vi "LOX_PID_screen_V2.5.vi"() -> ()   [LabVIEW 2022 SP3]
panel:
  out "Countdown Timer (CDT)":dbl format="T%<+%H:%M:%S%3u>t"
  out "Date":timestamp format="%<%d/%m/%Y>T"
  in  "Close":bool
  in  "Screen No":dbl
  out "Indian Standard Time (IST)":timestamp format="%<%H:%M:%S%2u>T"
  out "Boolean 77":bool
  out "B_GN_PV_01":bool caption="Boolean"
  out "Boolean 61":bool
  out "B_GN_PV_03":bool caption="Boolean"
  out "Boolean 76":bool
  out "B_GN_PV_04":bool caption="Boolean"
  out "Boolean 60":bool
  out "B_GN_PV_07":bool caption="Boolean"
  out "Boolean 73":bool
  out "B_LO_PV_02":bool caption="Boolean"
  out "B_GN_P_10":dbl format="%.2f bar"
  out "B_GN_P_09":dbl format="%.2f bar"
  out "B_GN_P_03":dbl format="%.2f bar"
  out "B_GN_CV_01":dbl format="%.0f %%"
  out "Boolean 59":bool
  out "B_GN_CV_01":bool caption="Boolean"
  out "B_GN_P_05":dbl format="%.2f bar"
  out "B_GN_P_04":dbl format="%.2f bar"
  out "B_GN_P_06":dbl format="%.2f bar"
  out "B_GN_P_32":dbl format="%.2f bar"
  out "Boolean 40":bool
  out "B_GN_PV_09":bool caption="Boolean"
  out "Boolean 41":bool
  out "B_GN_PV_08":bool caption="Boolean"
  out "B_GN_P_08":dbl format="%.2f bar"
  out "B_GN_P_07":dbl format="%.2f bar"
  out "B_GN_P_01":dbl format="%.2f bar"
  out "B_GO_P_04":dbl format="%.2f bar"
  out "B_GN_P_02":dbl format="%.2f bar"
  out "B_GN_P_12":dbl format="%.2f bar"
  out "B_GN_T_01":dbl format="%.2f bar"
  out "B_GN_P_11":dbl format="%.2f bar"
  out "B_GN_P_13":dbl format="%.2f bar"
  out "B_GO_P_03":dbl format="%.2f bar"
  out "B_GO_P_01":dbl format="%.2f bar"
  out "B_GO_P_02":dbl format="%.2f bar"
  out "B_GN_P_33":dbl format="%.2f bar"
  out "Boolean 74":bool
  out "B_LO_PV_09":bool caption="Boolean"
  out "Boolean 63":bool
  out "B_LO_PV":bool caption="Boolean"
  out "Boolean 66":bool
  out "B_LO_PV_13":bool caption="Boolean"
  out "Boolean 67":bool
  out "B_LO_PV_05":bool caption="Boolean"
  out "Boolean 65":bool
  out "B_LO_PV_06":bool caption="Boolean"
  out "B_LO_P_10":dbl format="%.2f bar"
  out "B_LO_FM_02":dbl format="%.2f Kg/s"
  out "Boolean 68":bool
  out "B_LO_PV_04":bool caption="Boolean"
  out "Boolean 75":bool
  out "B_LO_PV_12":bool caption="Boolean"
  out "Boolean 64":bool
  out "B_LO_PV_10":bool caption="Boolean"
  out "Boolean 62":bool
  out "B_LO_PV_11":bool caption="Boolean"
  out "B_LO_P_06":dbl format="%.2f bar"
  out "B_LO_T_06":dbl format="%.2f bar"
  out "Boolean 71":bool
  out "B_LO_PV_07":bool caption="Boolean"
  out "Boolean 69":bool
  out "B_LO_PV_08":bool caption="Boolean"
  out "B_LO_P_03":dbl format="%.2f bar"
  out "B_LO_T_03":dbl format="%.2f bar"
  out "B_LO_FM_03":dbl format="%.2f Kg/s"
  out "B_LO_P_09":dbl format="%.2f bar"
  out "Boolean 70":bool
  out "B_LO_PV_03":bool caption="Boolean"
  out "B_LO_P_08":dbl format="%.2f bar"
  out "B_LO_P_01":dbl format="%.2f bar"
  out "B_LO_T_01":dbl format="%.2f bar"
  out "Boolean 72":bool
  out "B_LO_PV_02":bool caption="Boolean"
  out "B_LO_P_02":dbl format="%.2f bar"
  out "B_LO_P_07":dbl format="%.2f bar"
  out "B_LO_T_02":dbl format="%.2f bar"
  out "B_LO_P_11":dbl format="%.2f bar"
  out "B_LN_T_03":dbl format="%.2f bar"
  out "B_LN_P_08":dbl format="%.2f bar"
  out "B_LO_P_05":dbl format="%.2f bar"
  out "B_LO_P_04":dbl format="%.2f bar"
  out "B_LO_T_04":dbl format="%.2f bar"
  out "B_LO_T_05":dbl format="%.2f bar"
  out "B_HE_P_03":dbl format="%.2f bar"
  out "B_HE_T_01":dbl format="%.2f bar"
  out "B_HE_P_04":dbl format="%.2f bar"
  out "B_HE_T_03":dbl format="%.2f bar"
  out "B_HE_T_02":dbl format="%.2f bar"
  out "B_HE_P_02":dbl format="%.2f bar"
  out "B_HE_P_01":dbl format="%.2f bar"
  out "B_LO_FM_01":dbl format="%.2f Kg/s"
  # "BSTF P&ID SCREEN"
  # "VERSION 2.1"
  # "Stage Cryo Valves Command"
  # "Connect to all stage LOX and LIN EV"
  # "Connect to all ground LOX and LIN EV"
  # "LOX/LIN Ground Valves Command"
  # "GOX Ignitor Purge"
  # "Engine LOX Injector Purge"
  # "To Atmosphere"
  # "LOX/LIN Feed Line Purge"
  # "Connected to\nStage COPV \nUbmilical"
  # "LOX Tank Pressurization"
  # "LOX Tank\nVent"
  # "GHe\nSource"
  # "LOX PUMP SEAL PURGE"
  # "ENGINE"
  # "GOX IGNITOR PURGE"
  # "CommonGN2\nSource"
  # "GN2\nVaporisr\nSource"
  # "GOX\nSource"
  # "LOX\nSource"
  # "GOX MANIFOLD"
  # "B_LO_SP_01"
  # "LOX\n31KL\nTANK"
  # "BOOSTER PUMP"
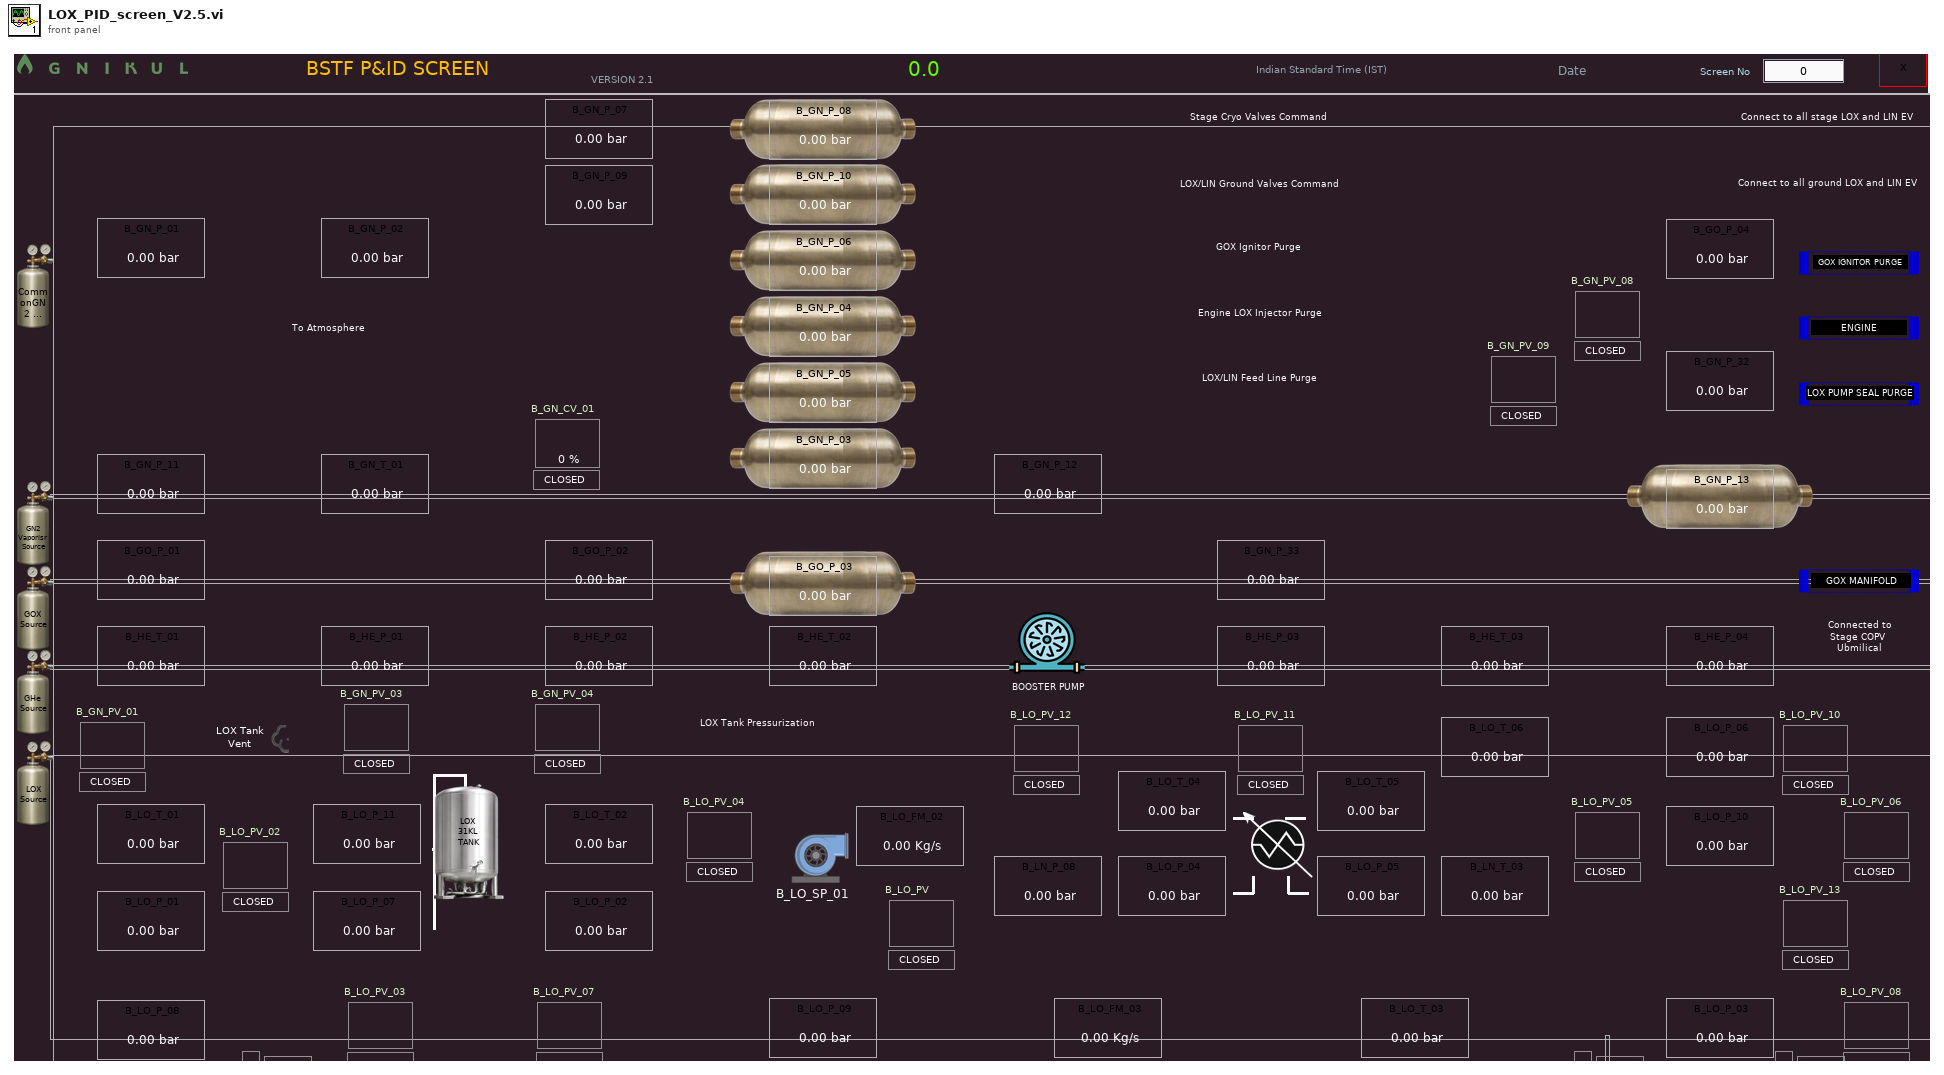
[diagram p1: front panel]
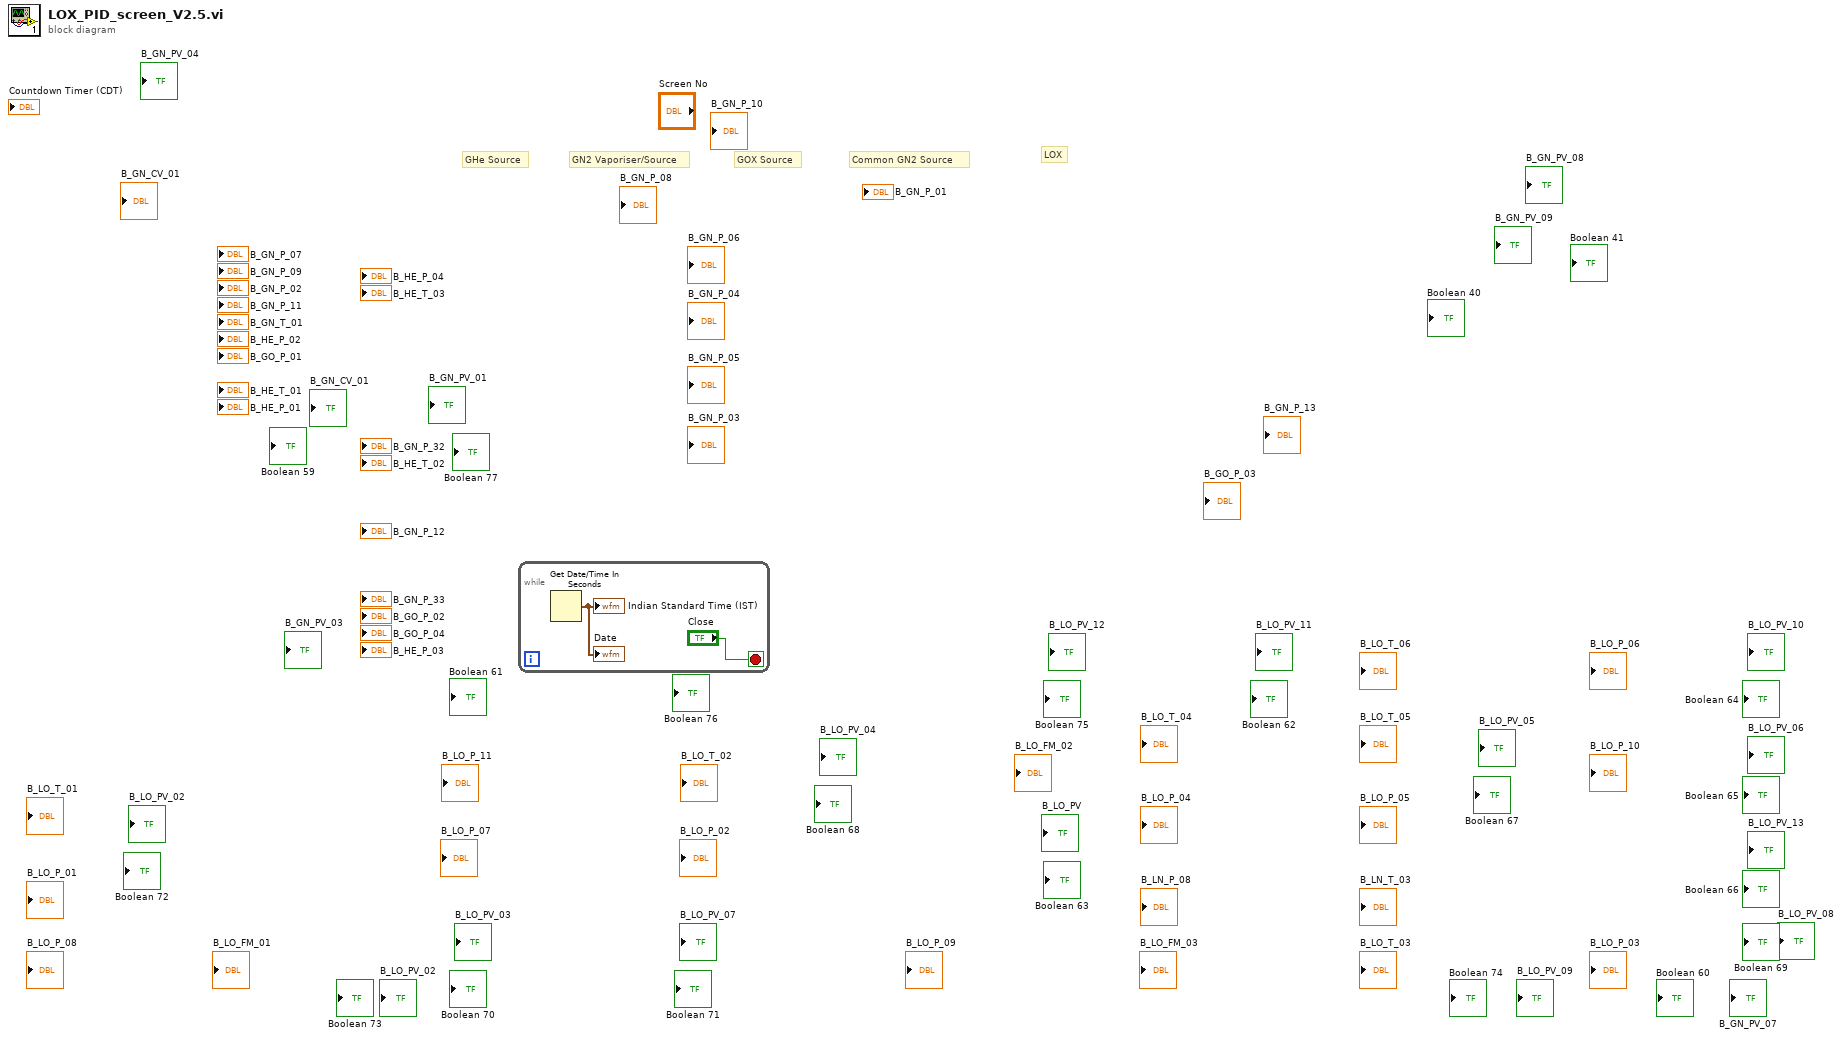
[diagram p0: block diagram]
diagram:
  # "LOX"
  # "Common GN2 Source"
  # "GOX Source"
  # "GN2 Vaporiser/Source"
  # "GHe Source"
  n1 = while {
    stop <- "Close" stop-if-true
    n2 = Get Date/Time In Seconds() -> (seconds since 1Jan1904=→"Date" →"Indian Standard Time (IST)":timestamp)
  }
